vi "UHR-Fleezers Control (host) - 10.3.vi"() -> ()   [LabVIEW 2010] (continued)
          tunnel: w7743 -> [w7751]
          tunnel: w7741 -> [w7750]
          tunnel: w7740 -> [w7749]
          tunnel: [w7748] -> w7739
          tunnel: [w7747] -> w7738
          tunnel: ["Cap 1 Samp Flow ON"] -> w7737
          tunnel: w7739 -> [w7775]
          tunnel: w7738 -> [w7774]
          tunnel: w7737 -> [w7773]
          frame #0 {
            n1615 = local read "Saved Stage Positions"() -> (w7762:dbl[][])
            n1616 = Array Subset(array=w7762, index (row)=0 ("index"), length (row)=1 ("length"), index (col)=1 ("index"), length (col)=3 ("length")) -> (w7759:dbl[][])
            n1617 = Reshape Array(w7759, 3 ("dimension size")) -> (w7757:dbl[])
            n1618 = Array To Cluster(array=w7757) -> (cluster=w7756:cluster{"[0]":dbl, "[1]":dbl, "[2]":dbl})
            n1619 = case shown="True" "Cap 1 Samp Flow ON" {
              tunnel: w7749 -> [w7764 w7770]
              tunnel: w7750 -> [w7765 w7769]
              tunnel: [w7765 w7767] -> w7748
              tunnel: [w7764 w7766] -> w7747
              frame False {
              }
              frame True {
                # "run flow"
                n1620 = Concatenate Strings("run" ("string"), "\r") -> (w7771:string)
                n1621 = VISA Write(VISA resource name=w7769, write buffer=w7771, error in (no error)=w7770) -> (VISA resource name out=w7767:refnum<visa-resource-name>, error out=w7766:errorcluster)  [unwired: 1 out]
              }
            }
            n1622 = call "Set Stage Position.vi"("Position"=w7756, "error in"=w7751, "VISA resource name in"=w7752) -> ("error out"=w7755:errorcluster)  [unwired: 2 out]
            n1623 = local write "Stage Control Serial Error"(w7755) -> ()
            n1624 = local write "Stage Moving"(TRUE ("Stage Moving")) -> ()
          }
          frame #1 {
            n1625 = local write "Stage Moving"(FALSE ("Stage Moving")) -> ()
            n1626 = case shown="True" w7773 {
              tunnel: w7774 -> [w7780 w7786]
              tunnel: w7775 -> [w7781 w7785]
              tunnel: [w7781 w7783] -> _
              tunnel: [w7780 w7782] -> _
              frame False {
              }
              frame True {
                n1627 = Concatenate Strings("stop" ("string"), "\r") -> (w7787:string)
                n1628 = VISA Write(VISA resource name=w7785, write buffer=w7787, error in (no error)=w7786) -> (VISA resource name out=w7783:refnum<visa-resource-name>, error out=w7782:errorcluster)  [unwired: 1 out]
              }
            }
            n1629 = case shown="True" TRUE {
              tunnel: "Cap 1 T ON" -> [w7790 w7791]
              frame False {
                n1630 = property on="Trap 1 (ON/OFF)" class="Bool (strict)"("Val(Sgnl)"=w7790) -> ()  [unwired: 2 in, 2 out]
              }
              frame True {
                n1631 = property on="Trap 2 (ON/OFF)" class="Bool (strict)"("Val(Sgnl)"=w7791) -> ()  [unwired: 2 in, 2 out]
              }
            }
            n1632 = call <vilib>:"Beep.vi"() -> ()  [unwired: 3 in, 9 out]
            n1633 = case shown="True" "Cap 1 Flow ON" {
              frame False {
              }
              frame True {
                n1634 = property on="Inject Pump 1" class="Bool (strict)"("Val(Sgnl)"=TRUE ("Value (Signaling)")) -> ()  [unwired: 2 in, 2 out]
              }
            }
          }
        }
      }
      event "Move Cap. 2 (ADig Left)": Value Change {
        n1635 = event-data() -> ()  [unwired: 1 in, 5 out]
        n1636 = local write "Move Cap. 2 (ADig Left)"(FALSE ("Move Cap. 2 (ADig Left)")) -> ()
        n1637 = flat-sequence {
          tunnel: w7799 -> [w7807]
          tunnel: w7798 -> [w7806]
          tunnel: w7796 -> [w7805]
          tunnel: w7795 -> [w7804]
          tunnel: [w7803] -> w7794
          tunnel: [w7802] -> w7793
          tunnel: ["Cap 2 Samp Flow ON"] -> w7792
          tunnel: w7794 -> [w7830]
          tunnel: w7793 -> [w7829]
          tunnel: w7792 -> [w7828]
          frame #0 {
            n1638 = local read "Saved Stage Positions"() -> (w7817:dbl[][])
            n1639 = case shown="True" "Cap 2 Samp Flow ON" {
              tunnel: w7805 -> [w7819 w7825]
              tunnel: w7804 -> [w7820 w7824]
              tunnel: [w7820 w7822] -> w7803
              tunnel: [w7819 w7821] -> w7802
              frame False {
              }
              frame True {
                # "run flow"
                n1640 = Concatenate Strings("run" ("string"), "\r") -> (w7826:string)
                n1641 = VISA Write(VISA resource name=w7824, write buffer=w7826, error in (no error)=w7825) -> (VISA resource name out=w7822:refnum<visa-resource-name>, error out=w7821:errorcluster)  [unwired: 1 out]
              }
            }
            n1642 = Array Subset(array=w7817, index (row)=1 ("index"), length (row)=1 ("length"), index (col)=1 ("index"), length (col)=3 ("length")) -> (w7814:dbl[][])
            n1643 = Reshape Array(w7814, 3 ("dimension size")) -> (w7812:dbl[])
            n1644 = Array To Cluster(array=w7812) -> (cluster=w7811:cluster{"[0]":dbl, "[1]":dbl, "[2]":dbl})
            n1645 = call "Set Stage Position.vi"("Position"=w7811, "error in"=w7806, "VISA resource name in"=w7807) -> ("error out"=w7810:errorcluster)  [unwired: 2 out]
            n1646 = local write "Stage Moving"(TRUE ("Stage Moving")) -> ()
            n1647 = local write "Stage Control Serial Error"(w7810) -> ()
          }
          frame #1 {
            n1648 = local write "Stage Moving"(FALSE ("Stage Moving")) -> ()
            n1649 = case shown="True" TRUE {
              tunnel: "Cap 2 T ON" -> [w7841 w7842]
              frame False {
                n1650 = property on="Trap 2 (ON/OFF)" class="Bool (strict)"("Val(Sgnl)"=w7841) -> ()  [unwired: 2 in, 2 out]
              }
              frame True {
                n1651 = property on="Trap 1 (ON/OFF)" class="Bool (strict)"("Val(Sgnl)"=w7842) -> ()  [unwired: 2 in, 2 out]
              }
            }
            n1652 = call <vilib>:"Beep.vi"() -> ()  [unwired: 3 in, 9 out]
            n1653 = case shown="True" w7828 {
              tunnel: w7830 -> [_ w7836]
              tunnel: w7829 -> [_ w7835]
              frame False {
              }
              frame True {
                n1654 = Concatenate Strings("stop" ("string"), "\r") -> (w7838:string)
                n1655 = VISA Write(VISA resource name=w7836, write buffer=w7838, error in (no error)=w7835) -> ()  [unwired: 3 out]
              }
            }
            n1656 = case shown="True" "Cap 2 Flow ON" {
              frame False {
              }
              frame True {
                n1657 = property on="Inject Pump 3" class="Bool (strict)"("Val(Sgnl)"=TRUE ("Value (Signaling)")) -> ()  [unwired: 2 in, 2 out]
              }
            }
          }
        }
      }
      event "+z", "-z": Value Change {
        n1658 = event-data() -> ()  [unwired: 1 in, 5 out]
        n1659 = flat-sequence {
          tunnel: w7843 -> [w7865]
          tunnel: w7844 -> [w7845]
          frame #0 {
            n1660 = call "Read Stage Position.vi"("error in"=w7865, "VISA resource name in"=w7845) -> ("Current Position"=w7850:cluster{dbl, dbl, dbl}, "error out"=w7863:errorcluster, "VISA resource name out"=w7864:refnum<visa-resource-name>)  [unwired: 1 out]
            n1661 = local read "Saved Stage Positions"() -> (w7874:dbl[][])
            n1662 = Divide(x="z nudge increment (um)", y=1000.0) -> (x/y=w7862:dbl)
            n1663 = Boolean To (0,1)(Boolean="+z") -> (0, 1=w7854:i16)
            n1664 = Boolean To (0,1)(Boolean="-z") -> (0, 1=w7855:i16)
            n1665 = Array Subset(array=w7874, index (row)=1 ("index"), length (row)=1 ("length"), index (col)=1 ("index"), length (col)=3 ("length")) -> (w7871:dbl[][])
            n1666 = Multiply(x=w7854, y=w7862) -> (x*y=w7858:dbl)
            n1667 = Multiply(x=w7855, y=w7862) -> (x*y=w7856:dbl)
            n1668 = Unbundle(w7850) -> (w7848:dbl, w7847:dbl, w7851:dbl)
            n1669 = Negate(x=w7856) -> (-x=w7857:dbl)
            n1670 = Reshape Array(w7871, 3 ("dimension size")) -> (w7869:dbl[])
            n1671 = Add(x=w7858, y=w7857) -> (x+y=w7859:dbl)
            n1672 = Array To Cluster(array=w7869) -> ()  [unwired: 1 out]
            n1673 = Add(x=w7859, y=w7851) -> (x+y=w7849:dbl)
            n1674 = Bundle(cluster=w7850, w7848, w7847, w7849) -> (w7846:cluster{dbl, dbl, dbl})
            n1675 = call "Set Stage Position.vi"("Position"=w7846, "error in"=w7863, "VISA resource name in"=w7864) -> ("error out"=w7868:errorcluster)  [unwired: 2 out]
            n1676 = local write "Stage Moving"(TRUE ("Stage Moving")) -> ()
            n1677 = local write "Stage Control Serial Error"(w7868) -> ()
          }
          frame #1 {
            n1678 = local write "Stage Moving"(FALSE ("Stage Moving")) -> ()
            n1679 = call <vilib>:"Beep.vi"() -> ()  [unwired: 3 in, 9 out]
          }
        }
      }
      event "Cal/Data Acq. Spot": Value Change {
        # "CALIBRATE DATA ACQUISITION SPOT? LOCATE WHERE TO COLLECT FLUORESCENCE FROM?"
        n1680 = event-data() -> ()  [unwired: 1 in, 5 out]
        n1681 = flat-sequence {
          tunnel: w7880 -> [w7883]
          tunnel: w7879 -> [w7882]
          tunnel: ["Cal @ (MHz)"] -> w7877
          tunnel: w7877 -> [w7903]
          tunnel: w7877 -> [w7924]
          frame #0 {
            n1682 = local read "Saved Stage Positions"() -> (w7886:dbl[][])
            n1683 = Array Subset(array=w7886, index (row)=2 ("index"), length (row)=1 ("length"), index (col)=1 ("index"), length (col)=3 ("length")) -> (w7889:dbl[][])
            n1684 = Reshape Array(w7889, 3 ("dimension size")) -> (w7891:dbl[])
            n1685 = local write "Stage Moving"(TRUE ("Stage Moving")) -> ()
            n1686 = Array To Cluster(array=w7891) -> (cluster=w7892:cluster{"[0]":dbl, "[1]":dbl, "[2]":dbl})
            n1687 = call "Set Stage Position.vi"("Position"=w7892, "error in"=w7882, "VISA resource name in"=w7883) -> ("error out"=w7893:errorcluster)  [unwired: 2 out]
            n1688 = local write "Stage Control Serial Error"(w7893) -> ()
          }
          frame #1 {
            n1689 = property on="Trap Delta (MHz)" class="DigNum (strict)"("Val(Sgnl)"="Cal @ (MHz)") -> ()  [unwired: 2 in, 2 out]
            n1690 = local write "Stage Moving"(FALSE ("Stage Moving")) -> ()
            n1691 = call <vilib>:"Beep.vi"() -> ()  [unwired: 3 in, 9 out]
          }
          frame #2 {
            n1692 = Wait (ms)(milliseconds to wait=u32 100) -> ()  [unwired: 1 out]
          }
          frame #3 {
            n1693 = property on="Save Calibration" class="Bool (strict)"("Val(Sgnl)"=TRUE ("Value (Signaling)")) -> ()  [unwired: 2 in, 2 out]
          }
          frame #4 {
            n1694 = Wait (ms)(milliseconds to wait=u32 4000) -> ()  [unwired: 1 out]
          }
          frame #5 {
            n1695 = while {
              stop <- w7900 stop-if-true
              n1696 = local read "Saving..."() -> (w7901:bool)
              n1697 = Wait (ms)(milliseconds to wait=u32 100) -> ()  [unwired: 1 out]
              n1698 = Not(x=w7901) -> (.not. x?=w7900:bool)
            }
          }
          frame #6 {
            n1699 = case shown="True" "W/ Offset 1" {
              tunnel: w7903 -> [_ w7905]
              frame False {
              }
              frame True {
                n1700 = stacked-sequence {
                  tunnel: w7905 -> [_ _ _ _ _ _ _ w7922]
                  frame #0 {
                    n1701 = property on="Trap Delta (MHz)" class="DigNum (strict)"("Val(Sgnl)"="Offset 1 Start (MHz)") -> ()  [unwired: 2 in, 2 out]
                    n1702 = Replace Array Subset(array=u32[] [0] ("Index Values"), new element="Offset 1 Set", index=0) -> (w7906:u32[])
                    n1703 = property on="Saved AOD Raster Scan Parameter Sets" class="Arr (strict)"("Index Values"=w7906) -> ()  [unwired: 2 in, 2 out]
                  }
                  frame #1 {
                    n1704 = Wait (ms)(milliseconds to wait=u32 200) -> ()  [unwired: 1 out]
                  }
                  frame #2 {
                    n1705 = property on="Load parameters" class="Bool (strict)"("Val(Sgnl)"=TRUE ("Value (Signaling)")) -> ()  [unwired: 2 in, 2 out]
                  }
                  frame #3 {
                    n1706 = Wait (ms)(milliseconds to wait=u32 200) -> ()  [unwired: 1 out]
                  }
                  frame #4 {
                    n1707 = property on="Trap Raster Scan" class="Bool (strict)"("Val(Sgnl)"=TRUE ("Value (Signaling)")) -> ()  [unwired: 2 in, 2 out]
                  }
                  frame #5 {
                    n1708 = Wait (ms)(milliseconds to wait=u32 2000) -> ()  [unwired: 1 out]
                  }
                  frame #6 {
                    n1709 = while {
                      stop <- w7919 stop-if-true
                      n1710 = local read "Raster Scanning..."() -> (w7921:bool)
                      n1711 = local read "Saving..."() -> (w7917:bool)
                      n1712 = Wait (ms)(milliseconds to wait=u32 100) -> ()  [unwired: 1 out]
                      n1713 = Not(x=w7917) -> (.not. x?=w7916:bool)
                      n1714 = Not(x=w7921) -> (.not. x?=w7918:bool)
                      n1715 = And(x=w7918, y=w7916) -> (x .and. y?=w7919:bool)
                    }
                  }
                  frame #7 {
                    n1716 = property on="Trap Delta (MHz)" class="DigNum (strict)"("Val(Sgnl)"=w7922) -> ()  [unwired: 2 in, 2 out]
                  }
                }
              }
            }
          }
          frame #7 {
            n1717 = local read "Save ave N"() -> (w7923:dbl)
            n1718 = case shown="True" "W/ Offset 2" {
              tunnel: w7924 -> [_ w7930]
              tunnel: w7923 -> [_ w7929]
              frame False {
                n1719 = Multiply(x="Cal read wait (s)", y=u32 1000 ("milliseconds to wait")) -> (x*y=w7927:u32)
                n1720 = Wait (ms)(milliseconds to wait=w7927) -> ()  [unwired: 1 out]
              }
              frame True {
                n1721 = stacked-sequence {
                  tunnel: w7930 -> [_ _ _ _ _ _ _ _ _ w7951 _ _]
                  tunnel: w7929 -> [_ _ _ _ _ _ _ _ _ w7949 _ _]
                  frame #0 {
                    n1722 = property on="Save ave N" class="DigNum (strict)"("Val(Sgnl)"=1.0 ("Value (Signaling)")) -> ()  [unwired: 2 in, 2 out]
                  }
                  frame #1 {
                    n1723 = Wait (ms)(milliseconds to wait=u32 500) -> ()  [unwired: 1 out]
                  }
                  frame #2 {
                    n1724 = property on="Trap Delta (MHz)" class="DigNum (strict)"("Val(Sgnl)"="Offset 2 Start (MHz)") -> ()  [unwired: 2 in, 2 out]
                    n1725 = Replace Array Subset(array=u32[] [0] ("Index Values"), new element="Offset 2 Set", index=0) -> (w7935:u32[])
                    n1726 = property on="Saved AOD Raster Scan Parameter Sets" class="Arr (strict)"("Index Values"=w7935) -> ()  [unwired: 2 in, 2 out]
                  }
                  frame #3 {
                    n1727 = Wait (ms)(milliseconds to wait=u32 500) -> ()  [unwired: 1 out]
                  }
                  frame #4 {
                    n1728 = property on="Load parameters" class="Bool (strict)"("Val(Sgnl)"=TRUE ("Value (Signaling)")) -> ()  [unwired: 2 in, 2 out]
                  }
                  frame #5 {
                    n1729 = Wait (ms)(milliseconds to wait=u32 500) -> ()  [unwired: 1 out]
                  }
                  frame #6 {
                    n1730 = property on="Trap Raster Scan" class="Bool (strict)"("Val(Sgnl)"=TRUE ("Value (Signaling)")) -> ()  [unwired: 2 in, 2 out]
                  }
                  frame #7 {
                    n1731 = Wait (ms)(milliseconds to wait=u32 2000) -> ()  [unwired: 1 out]
                  }
                  frame #8 {
                    n1732 = while {
                      stop <- w7944 stop-if-true
                      n1733 = local read "Raster Scanning..."() -> (w7947:bool)
                      n1734 = local read "Saving..."() -> (w7945:bool)
                      n1735 = Wait (ms)(milliseconds to wait=u32 100) -> ()  [unwired: 1 out]
                      n1736 = Not(x=w7945) -> (.not. x?=w7943:bool)
                      n1737 = Not(x=w7947) -> (.not. x?=w7946:bool)
                      n1738 = And(x=w7946, y=w7943) -> (x .and. y?=w7944:bool)
                    }
                  }
                  frame #9 {
                    n1739 = property on="Trap Delta (MHz)" class="DigNum (strict)"("Val(Sgnl)"=w7951) -> ()  [unwired: 2 in, 2 out]
                    n1740 = property on="Saved AOD Raster Scan Parameter Sets" class="Arr (strict)"("Index Values"=u32[] [0]) -> ()  [unwired: 2 in, 2 out]
                    n1741 = property on="Save ave N" class="DigNum (strict)"("Val(Sgnl)"=w7949) -> ()  [unwired: 2 in, 2 out]
                  }
                  frame #10 {
                    n1742 = Wait (ms)(milliseconds to wait=u32 500) -> ()  [unwired: 1 out]
                  }
                  frame #11 {
                    n1743 = property on="Load parameters" class="Bool (strict)"("Val(Sgnl)"=TRUE ("Value (Signaling)")) -> ()  [unwired: 2 in, 2 out]
                  }
                }
              }
            }
          }
          frame #8 {
            n1744 = property on="Read Cal" class="Bool (strict)"("Val(Sgnl)"=TRUE ("Value (Signaling)")) -> ()  [unwired: 2 in, 2 out]
          }
          frame #9 {
            n1745 = Wait (ms)(milliseconds to wait=u32 500) -> ()  [unwired: 1 out]
          }
          frame #10 {
            n1746 = property on="Fish for Tether" class="Bool (strict)"("Val(Sgnl)"=TRUE ("Value (Signaling)")) -> ()  [unwired: 2 in, 2 out]
          }
        }
        n1747 = local write "Cal/Data Acq. Spot"(FALSE ("Cal/Data Acq. Spot")) -> ()
      }
      event "Dump Beads": Value Change {
        # "SCRIPT TO REMOVE BOTH BEADS FROM THE TRAPS. TURNS ON LIGHT WHICH INDICATES THAT STAGE IS MOVING. THEN STOPS SAVING DATA. \nSETS Sample Channel Flow TO TRUE. STOPS INTERLACING GREEN FLUORESCENCE. TURNS OFF Tether INDICATOR BECAUSE WE ARE THROWING IT\nAWAY. SHUTS OFF TRAP POSITION FEEDBACK."
        n1748 = event-data() -> ()  [unwired: 1 in, 5 out]
        n1749 = flat-sequence {
          tunnel: w7958 -> [w7964]
          tunnel: w7957 -> [w7963]
          frame #0 {
            w7960 = FALSE ("Fl. Triggered...")
            w7961 = TRUE ("Stage Moving")
            n1750 = local read "Saving..."() -> (w7962:bool)
            n1751 = local write "Fl. Triggered..."(w7960) -> ()
            n1752 = local write "Stage Moving"(w7961) -> ()
            n1753 = local write "Tether"(w7960) -> ()
            n1754 = property on="Green Laser ON/Interlacing" class="Bool (strict)"("Val(Sgnl)"=w7960) -> ()  [unwired: 2 in, 2 out]
            n1755 = property on="Trap Pos. FB ON" class="Bool (strict)"("Val(Sgnl)"=w7960) -> ()  [unwired: 2 in, 2 out]
            n1756 = property on="Sample Channel Flow" class="Bool (strict)"("Val(Sgnl)"=w7961) -> ()  [unwired: 2 in, 2 out]
            n1757 = local write "Stop Saving"(w7962) -> ()
          }
          frame #1 {
            # "MOVES TO THE DUMP BEADS POSITION"
            n1758 = local read "Saved Stage Positions"() -> (w7965:dbl[][])
            n1759 = Array Subset(array=w7965, index (row)=3 ("index"), length (row)=1 ("length"), index (col)=1 ("index"), length (col)=3 ("length")) -> (w7970:dbl[][])
            n1760 = Reshape Array(w7970, 3 ("dimension size")) -> (w7968:dbl[])
            n1761 = Array To Cluster(array=w7968) -> (cluster=w7967:cluster{"[0]":dbl, "[1]":dbl, "[2]":dbl})
            n1762 = call "Set Stage Position.vi"("Position"=w7967, "error in"=w7963, "VISA resource name in"=w7964) -> ()  [unwired: 3 out]
          }
          frame #2 {
            w7974 = FALSE ("Value (Signaling)")
            # "TURNS TRAPS OFF SO THAT\nBEADS REMAIN AT DUMP \nBEADS POSITION"
            n1763 = property on="Trap 1 (ON/OFF)" class="Bool (strict)"("Val(Sgnl)"=w7974) -> ()  [unwired: 2 in, 2 out]
            n1764 = property on="Trap 2 (ON/OFF)" class="Bool (strict)"("Val(Sgnl)"=w7974) -> ()  [unwired: 2 in, 2 out]
            n1765 = call <vilib>:"Beep.vi"() -> ()  [unwired: 3 in, 9 out]
          }
          frame #3 {
            # "MOVES STAGE BACK TO THE\nANTIDIG CAPILARY BY CALLING\nTHE Move Cap. 2 SCRIPT"
            n1766 = property on="Move Cap. 2 (ADig Left)" class="Bool (strict)"("Val(Sgnl)"=TRUE ("Value (Signaling)")) -> ()  [unwired: 2 in, 2 out]
          }
        }
      }
      event "Dip for Protein": Value Change {
        n1767 = event-data() -> ()  [unwired: 1 in, 5 out]
        n1768 = flat-sequence {
          tunnel: w7982 -> [w7986]
          tunnel: w7983 -> [w7987]
          tunnel: [w7987] -> w7977
          tunnel: [w7986] -> w7976
          tunnel: [w7990] -> w7980
          tunnel: [w7989] -> w7978
          tunnel: w7977 -> [w7993]
          tunnel: w7976 -> [w7992]
          tunnel: [w8003] -> w7981
          tunnel: w7980 -> [w8003]
          tunnel: [w8002] -> w7979
          tunnel: w7978 -> [w8002]
          tunnel: w7981 -> [w8008]
          tunnel: w7979 -> [w8007]
          frame #0 {
            n1769 = case shown="True" "Move Trap Before?" {
              frame False {
              }
              frame True {
                n1770 = property on="Trap Delta (MHz)" class="DigNum (strict)"("Val(Sgnl)"="Dip Trap Delta 1 (MHz)") -> ()  [unwired: 2 in, 2 out]
              }
            }
          }
          frame #1 {
            n1771 = local read "Saved Stage Positions"() -> (w7991:dbl[][])
            n1772 = Array Subset(array=w7991, index (row)=4 ("index"), length (row)=1 ("length"), index (col)=1 ("index"), length (col)=3 ("length")) -> (w7998:dbl[][])
            n1773 = Reshape Array(w7998, 3 ("dimension size")) -> (w7996:dbl[])
            n1774 = Array To Cluster(array=w7996) -> (cluster=w7995:cluster{"[0]":dbl, "[1]":dbl, "[2]":dbl})
            n1775 = call "Set Stage Position.vi"("Position"=w7995, "error in"=w7992, "VISA resource name in"=w7993) -> ("error out"=w7989:errorcluster, "VISA resource name out"=w7990:refnum<visa-resource-name>)  [unwired: 1 out]
          }
          frame #2 {
            n1776 = Multiply(x="Duration (s)", y=1000.0) -> (x*y=w8004:dbl)
            n1777 = Wait (ms)(milliseconds to wait=w8004) -> ()  [unwired: 1 out]
          }
          frame #3 {
            n1778 = local read "Saved Stage Positions"() -> (w8009:dbl[][])
            n1779 = Array Subset(array=w8009, index (row)=2 ("index"), length (row)=1 ("length"), index (col)=1 ("index"), length (col)=3 ("length")) -> (w8014:dbl[][])
            n1780 = Reshape Array(w8014, 3 ("dimension size")) -> (w8012:dbl[])
            n1781 = Array To Cluster(array=w8012) -> (cluster=w8011:cluster{"[0]":dbl, "[1]":dbl, "[2]":dbl})
            n1782 = call "Set Stage Position.vi"("Position"=w8011, "error in"=w8007, "VISA resource name in"=w8008) -> ()  [unwired: 3 out]
          }
          frame #4 {
            n1783 = case shown="True" "Move Trap After?" {
              frame False {
              }
              frame True {
                n1784 = property on="Trap Delta (MHz)" class="DigNum (strict)"("Val(Sgnl)"="Dip Trap Delta 2 (MHz)") -> ()  [unwired: 2 in, 2 out]
              }
            }
          }
          frame #5 {
            n1785 = case shown="True" "Green ON After?" {
              frame False {
              }
              frame True {
                n1786 = property on="Green Laser ON/Interlacing" class="Bool (strict)"("Val(Sgnl)"=TRUE ("Value (Signaling)")) -> ()  [unwired: 2 in, 2 out]
              }
            }
          }
          frame #6 {
            n1787 = Wait (ms)(milliseconds to wait=u32 500) -> ()  [unwired: 1 out]
          }
          frame #7 {
            n1788 = case shown="True" "Save Data After?" {
              frame False {
              }
              frame True {
                n1789 = property on="Start Saving" class="Bool (strict)"("Val(Sgnl)"=TRUE ("Value (Signaling)")) -> ()  [unwired: 2 in, 2 out]
              }
            }
          }
        }
      }
      event "Profile": Value Change {
        n1790 = event-data() -> ()  [unwired: 1 in, 5 out]
        n1791 = flat-sequence {
          tunnel: w8033 -> [w8036]
          tunnel: w8032 -> [w8044]
          tunnel: [w8038] -> w8031
          tunnel: [w8037] -> w8030
          tunnel: [w8035] -> w8028
          tunnel: [w8034] -> w8025
          tunnel: w8031 -> [w8051]
          tunnel: w8030 -> [w8050]
          tunnel: [w8048] -> w8029
          tunnel: w8028 -> [w8049]
          tunnel: [w8047] -> w8027
          tunnel: [w8046] -> w8026
          tunnel: w8025 -> [w8046]
          tunnel: w8029 -> [w8055]
          tunnel: w8027 -> [w8054]
          tunnel: w8026 -> [w8053]
          frame #0 {
            n1792 = call "Read Stage Position.vi"("error in"=w8044, "VISA resource name in"=w8036) -> ("Current Position"=w8034:cluster{dbl, dbl, dbl}, "error out"=w8037:errorcluster, "VISA resource name out"=w8035:refnum<visa-resource-name>)  [unwired: 1 out]
            "Current Position" <- w8034
            n1793 = local write "Stage Control Serial Error"(w8037) -> ()
            n1794 = Unbundle(w8034) -> (w8041:dbl, w8043:dbl, w8039:dbl)
            n1795 = Add(x=w8043, y="Y change (mm)") -> (x+y=w8040:dbl)
            n1796 = Bundle(w8041, w8040, w8039) -> (w8038:cluster{dbl, dbl, dbl})  [unwired: 1 in]
          }
          frame #1 {
            # "move to new position and start saving"
            n1797 = local write "Stage Moving"(TRUE ("Stage Moving")) -> ()
            n1798 = local write "Start Saving"(TRUE ("Start Saving")) -> ()
            n1799 = call "Set Stage Position.vi"("Position"=w8051, "error in"=w8050, "VISA resource name in"=w8049) -> ("error out"=w8047:errorcluster, "VISA resource name out"=w8048:refnum<visa-resource-name>)  [unwired: 1 out]
          }
          frame #2 {
            # "go back to start"
            n1800 = call "Set Stage Position.vi"("Position"=w8053, "error in"=w8054, "VISA resource name in"=w8055) -> ()  [unwired: 3 out]
          }
          frame #3 {
            # "stop saving"
            n1801 = local write "Stop Saving"(TRUE ("Stop Saving")) -> ()
            n1802 = local write "Stage Moving"(FALSE ("Stage Moving")) -> ()
          }
        }
      }
      event "Move to Position 1", "Move to Position 2", "Move to Position 3", "Move to Position 4", "Move to Position 5", "Lower Ch. Cap.": Value Change {
        n1803 = event-data() -> ()  [unwired: 1 in, 5 out]
        n1804 = Or(x="Move to Position 5", y="Lower Ch. Cap.") -> (x .or. y?=w8061:bool)
        n1805 = Build Array("Move to Position 1", "Move to Position 2", "Move to Position 3", "Move to Position 4", w8061) -> (w8064:bool[])
        n1806 = Boolean Array To Number(Boolean array=w8064) -> (number=w8063:u32)
        n1807 = Logarithm Base 2(1:w8063) -> (0:w8062:dbl)
        n1808 = flat-sequence {
          tunnel: w8062 -> [w8073]
          tunnel: w8059 -> [w8071]
          tunnel: w8058 -> [w8070]
          frame #0 {
            n1809 = local read "Saved Stage Positions"() -> (w8081:dbl[][])
            n1810 = Array Subset(array=w8081, index (row)=w8073, length (row)=1 ("length"), index (col)=1 ("index"), length (col)=3 ("length")) -> (w8078:dbl[][])
            n1811 = Reshape Array(w8078, 3 ("dimension size")) -> (w8076:dbl[])
            n1812 = Array To Cluster(array=w8076) -> (cluster=w8075:cluster{"[0]":dbl, "[1]":dbl, "[2]":dbl})
            n1813 = call "Set Stage Position.vi"("Position"=w8075, "error in"=w8070, "VISA resource name in"=w8071) -> ("error out"=w8074:errorcluster)  [unwired: 2 out]
            n1814 = local write "Stage Moving"(TRUE ("Stage Moving")) -> ()
            n1815 = local write "Stage Control Serial Error"(w8074) -> ()
          }
          frame #1 {
            n1816 = local write "Stage Moving"(FALSE ("Stage Moving")) -> ()
            n1817 = call <vilib>:"Beep.vi"() -> ()  [unwired: 3 in, 9 out]
          }
        }
      }
      event "Got ADig bead": Value Change {
        n1818 = event-data() -> ()  [unwired: 1 in, 5 out]
        n1819 = property on="Move Cap. 1 (DNA Right)" class="Bool (strict)"("Val(Sgnl)"=TRUE ("Value (Signaling)")) -> ()  [unwired: 2 in, 2 out]
        n1820 = property on="Inject Pump 3" class="Bool (strict)"("Val(Sgnl)"=FALSE ("Value (Signaling)")) -> ()  [unwired: 2 in, 2 out]
      }
      event "Got DNA bead": Value Change {
        n1821 = event-data() -> ()  [unwired: 1 in, 5 out]
        n1822 = property on="Cal/Data Acq. Spot" class="Bool (strict)"("Val(Sgnl)"=TRUE ("Value (Signaling)")) -> ()  [unwired: 2 in, 2 out]
        n1823 = property on="Inject Pump 1" class="Bool (strict)"("Val(Sgnl)"=FALSE ("Value (Signaling)")) -> ()  [unwired: 2 in, 2 out]
      }
      event "Take Stepping Data": Value Change {
        n1824 = event-data() -> ()  [unwired: 1 in, 5 out]
        n1825 = local read "Save ave N"() -> (w8098:dbl)
        n1826 = flat-sequence {
          tunnel: w8098 -> [w8100]
          tunnel: [w8100] -> w8093
          tunnel: [w8102] -> w8094
          tunnel: w8093 -> [w8102]
          tunnel: [w8104] -> w8095
          tunnel: w8094 -> [w8104]
          tunnel: [w8107] -> w8096
          tunnel: w8095 -> [w8107]
          tunnel: [w8109] -> w8097
          tunnel: w8096 -> [w8109]
          tunnel: [w8111] -> w8091
          tunnel: w8097 -> [w8111]
          tunnel: w8091 -> [w8114]
          tunnel: [w8114] -> w8090
          tunnel: w8090 -> [w8115]
          tunnel: [w8115] -> w8092
          tunnel: w8092 -> [w8121]
          frame #0 {
            n1827 = property on="Save ave N" class="DigNum (strict)"("Val(Sgnl)"="Save ave factor") -> ()  [unwired: 2 in, 2 out]
          }
          frame #1 {
            n1828 = Wait (ms)(milliseconds to wait=u32 100) -> ()  [unwired: 1 out]
          }
          frame #2 {
            n1829 = local read "Offset 2 Start (MHz)"() -> (w8106:dbl)
            n1830 = property on="Saved AOD Raster Scan Parameter Sets" class="Arr (strict)"("Index Values"=u32[] [2]) -> ()  [unwired: 2 in, 2 out]
            n1831 = property on="Trap Delta (MHz)" class="DigNum (strict)"("Val(Sgnl)"=w8106) -> ()  [unwired: 2 in, 2 out]
          }
          frame #3 {
            n1832 = property on="Load parameters" class="Bool (strict)"("Val(Sgnl)"=TRUE ("Value (Signaling)")) -> ()  [unwired: 2 in, 2 out]
          }
          frame #4 {
            n1833 = Wait (ms)(milliseconds to wait=u32 100) -> ()  [unwired: 1 out]
          }
          frame #5 {
            n1834 = property on="Trap Raster Scan" class="Bool (strict)"("Val(Sgnl)"=TRUE ("Value (Signaling)")) -> ()  [unwired: 2 in, 2 out]
          }
          frame #6 {
            n1835 = Wait (ms)(milliseconds to wait=u32 1000) -> ()  [unwired: 1 out]
          }
          frame #7 {
            n1836 = while {
              stop <- w8118 stop-if-true
              n1837 = local read "Raster Scanning..."() -> (w8120:bool)
              n1838 = local read "Saving..."() -> (w8119:bool)
              n1839 = Not(x=w8119) -> (.not. x?=w8116:bool)
              n1840 = Not(x=w8120) -> (.not. x?=w8117:bool)
              n1841 = And(x=w8117, y=w8116) -> (x .and. y?=w8118:bool)
            }
          }
          frame #8 {
            n1842 = property on="Save ave N" class="DigNum (strict)"("Val(Sgnl)"=w8121) -> ()  [unwired: 2 in, 2 out]
          }
        }
      }
      event "Step Size (nm)": Value Change {
        n1843 = event-data() -> ()  [unwired: 1 in, 5 out]
        n1844 = flat-sequence {
          frame #0 {
            n1845 = property on="Saved AOD Raster Scan Parameter Sets" class="Arr (strict)"("Index Values"=u32[] [1]) -> ()  [unwired: 2 in, 2 out]
          }
          frame #1 {
            n1846 = Multiply(x="N Steps", y="Step Size (nm)") -> (x*y=w8123:dbl)
            n1847 = property on="Scan Speed AOD (nm/s) 2" class="DigNum (strict)"("Value"="Step Size (nm)") -> ()  [unwired: 2 in, 2 out]
            n1848 = property on="Step Size AOD (nm) 2" class="DigNum (strict)"("Value"="Step Size (nm)") -> ()  [unwired: 2 in, 2 out]
            n1849 = property on="Scan Range AOD (nm) 2" class="DigNum (strict)"("Value"=w8123) -> ()  [unwired: 2 in, 2 out]
          }
        }
      }
      event "Take Detection Laser\nImage": Value Change {
        n1850 = event-data() -> ()  [unwired: 1 in, 5 out]
        n1851 = flat-sequence {
          tunnel: [w8151] -> w8141
          tunnel: [w8150] -> w8134
          tunnel: [w8149] -> w8126
          tunnel: [w8154] -> w8142
          tunnel: w8141 -> [w8154]
          tunnel: [w8153] -> w8135
          tunnel: w8134 -> [w8153]
          tunnel: [w8152] -> w8127
          tunnel: w8126 -> [w8152]
          tunnel: [w8158] -> w8143
          tunnel: w8142 -> [w8158]
          tunnel: [w8157] -> w8136
          tunnel: w8135 -> [w8157]
          tunnel: [w8156] -> w8128
          tunnel: w8127 -> [w8156]
          tunnel: [w8164] -> w8144
          tunnel: w8143 -> [w8164]
          tunnel: [w8163] -> w8137
          tunnel: w8136 -> [w8163]
          tunnel: [w8162] -> w8129
          tunnel: w8128 -> [w8162]
          tunnel: [w8168] -> w8145
          tunnel: w8144 -> [w8168]
          tunnel: [w8167] -> w8138
          tunnel: w8137 -> [w8167]
          tunnel: [w8166] -> w8130
          tunnel: w8129 -> [w8166]
          tunnel: [w8172] -> w8146
          tunnel: w8145 -> [w8172]
          tunnel: [w8171] -> w8139
          tunnel: w8138 -> [w8171]
          tunnel: [w8170] -> w8131
          tunnel: w8130 -> [w8170]
          tunnel: [w8176] -> w8147
          tunnel: w8146 -> [w8176]
          tunnel: [w8175] -> w8140
          tunnel: w8139 -> [w8175]
          tunnel: [w8174] -> w8132
          tunnel: w8131 -> [w8174]
          tunnel: w8147 -> [w8182]
          tunnel: w8140 -> [w8181]
          tunnel: [w8179] -> w8133
          tunnel: w8132 -> [w8179]
          tunnel: w8133 -> [w8183]
          frame #0 {
            n1852 = local read "Green Laser ON/Interlacing"() -> (w8151:bool)
            n1853 = local read "Green laser mode"() -> (w8150:enum32{"Laser ON", "Laser OFF", "Interlace"})
            n1854 = local read "Green FB On/Off"() -> (w8149:bool)
          }
          frame #1 {
            n1855 = property on="Green FB On/Off" class="Bool (strict)"("Val(Sgnl)"=FALSE ("Value (Signaling)")) -> ()  [unwired: 2 in, 2 out]
          }
          frame #2 {
            n1856 = property on="Green Laser ON/Interlacing" class="Bool (strict)"("Val(Sgnl)"=TRUE ("Value (Signaling)")) -> ()  [unwired: 2 in, 2 out]
            n1857 = property on="Flip Green Filter" class="Bool (strict)"("Val(Sgnl)"=TRUE ("Value (Signaling)")) -> ()  [unwired: 2 in, 2 out]
            n1858 = property on="Green laser mode" class="RadioBtnsControl (strict)"("Val(Sgnl)"=enum32{"Laser ON", "Laser OFF", "Interlace"}."Laser ON" ("Value (Signaling)")) -> ()  [unwired: 2 in, 2 out]
          }
          frame #3 {
            n1859 = Wait (ms)(milliseconds to wait=u32 500) -> ()  [unwired: 1 out]
          }
          frame #4 {
            n1860 = property on="Confocal Image" class="Bool (strict)"("Val(Sgnl)"=TRUE ("Value (Signaling)")) -> ()  [unwired: 2 in, 2 out]
          }
          frame #5 {
            n1861 = Wait (ms)(milliseconds to wait=u32 2000) -> ()  [unwired: 1 out]
          }
          frame #6 {
            n1862 = while {
              stop <- w8177 stop-if-true
              n1863 = local read "Saving..."() -> (w8178:bool)
              n1864 = Not(x=w8178) -> (.not. x?=w8177:bool)
            }
          }
          frame #7 {
            n1865 = property on="Flip Green Filter" class="Bool (strict)"("Val(Sgnl)"=TRUE ("Value (Signaling)")) -> ()  [unwired: 2 in, 2 out]
            n1866 = property on="Green Laser ON/Interlacing" class="Bool (strict)"("Val(Sgnl)"=w8182) -> ()  [unwired: 2 in, 2 out]
            n1867 = property on="Green laser mode" class="RadioBtnsControl (strict)"("Val(Sgnl)"=w8181) -> ()  [unwired: 2 in, 2 out]
          }
          frame #8 {
            n1868 = property on="Green FB On/Off" class="Bool (strict)"("Val(Sgnl)"=w8183) -> ()  [unwired: 2 in, 2 out]
          }
        }
      }
      event "Stop All": Value Change {
        n1869 = event-data() -> ()  [unwired: 1 in, 5 out]
        n1870 = local read "Stop All"() -> (w8184:bool)
      }
    }
    n1871 = node-c288() -> ()  [unwired: 1 in, 1 out]
  }
  n1872 = timed-loop "Mouse control: trap position (AOM deflection), set confocal spot from image" {
    tunnel: [w8186] -> w155
    tunnel: w8 -> [w8185]
    timing: w51 -> [_]
    timing-out: [_] -> w50
    stop <- w8186 stop-if-true
    n1873 = node-c288() -> ()  [unwired: 2 out]
    n1874 = event shown="[0] \"Pane\": Mouse Down" {
      selector: _ -> [_ _]
      dyn-events: _ -> [_ _]
      timeout: _ -> [_ _]
      tunnel: w8185 -> [w8189 _]
      event Mouse Down {
        n1875 = event-data() -> ("Time"=w8191:u32, "Coords"=w8190:T7, "Button"=w8192:u16)  [unwired: 6 out]
        n1876 = case shown="3" w8192 {
          tunnel: w8191 -> [_ _ w8295]
          tunnel: w8190 -> [_ w8229 w8293]
          tunnel: w8189 -> [_ _ w8291]
          frame 0, Default {
          }
          frame 1 {
            n1877 = property on="APD 2" class="ImageControl"() -> ("Displayed Image Position"=w8199:cluster{"Left":i32, "Top":i32})  [unwired: 2 in, 2 out]
            n1878 = property on="APD 1" class="ImageControl"() -> ("Displayed Image Position"=w8228:cluster{"Left":i32, "Top":i32})  [unwired: 2 in, 2 out]
            n1879 = property on="Detection Laser X" class="ImageControl"() -> ("Displayed Image Position"=w8225:cluster{"Left":i32, "Top":i32})  [unwired: 2 in, 2 out]
            n1880 = property on="Detection Laser Y" class="ImageControl"() -> ("Displayed Image Position"=w8224:cluster{"Left":i32, "Top":i32})  [unwired: 2 in, 2 out]
            n1881 = property on="APD 2" class="ImageControl"() -> ("Displayed Image Size"=w8198:cluster{"Width":u32, "Height":u32})  [unwired: 2 in, 2 out]
            n1882 = property on="APD 1" class="ImageControl"() -> ("Displayed Image Size"=w8226:cluster{"Width":u32, "Height":u32})  [unwired: 2 in, 2 out]
            n1883 = property on="Detection Laser X" class="ImageControl"() -> ("Displayed Image Size"=w8227:cluster{"Width":u32, "Height":u32})  [unwired: 2 in, 2 out]
            n1884 = property on="Detection Laser Y" class="ImageControl"() -> ("Displayed Image Size"=w8223:cluster{"Width":u32, "Height":u32})  [unwired: 2 in, 2 out]
            n1885 = Unbundle By Name(w8198) -> ("Width"=w8195:u32, "Height"=w8194:u32)
            n1886 = Unbundle By Name(w8199) -> ("Left"=w8197:i32, "Top"=w8196:i32)
            n1887 = Unbundle By Name(w8226) -> ("Width"=w8220:u32, "Height"=w8219:u32)
            n1888 = Unbundle By Name(w8227) -> ("Width"=w8216:u32, "Height"=w8215:u32)
            n1889 = Unbundle By Name(w8223) -> ("Width"=w8212:u32, "Height"=w8211:u32)
            n1890 = Unbundle By Name(w8228) -> ("Left"=w8222:i32, "Top"=w8221:i32)
            n1891 = Unbundle By Name(w8225) -> ("Left"=w8218:i32, "Top"=w8217:i32)
            n1892 = Unbundle By Name(w8224) -> ("Left"=w8214:i32, "Top"=w8213:i32)
            n1893 = Bundle("Left"=w8197, "Top"=w8196, "Width"=w8195, "Height"=w8194) -> (w8193:T45)  [unwired: 1 in]
            n1894 = Bundle("Left"=w8222, "Top"=w8221, "Width"=w8220, "Height"=w8219) -> (w8210:T45)  [unwired: 1 in]
            n1895 = Bundle("Left"=w8218, "Top"=w8217, "Width"=w8216, "Height"=w8215) -> (w8209:T45)  [unwired: 1 in]
            n1896 = Bundle("Left"=w8214, "Top"=w8213, "Width"=w8212, "Height"=w8211) -> (w8208:T45)  [unwired: 1 in]
            n1897 = Build Cluster Array(w8193, w8210, w8209, w8208) -> (w8207:T46)
            n1898 = for {
              tunnel: w8229 -> [w8240]
              tunnel: w8207 -> [w8241] mode=indexing
              shift-right: [w8238] -> w8205
              shift-left: TRUE -> [w8239]
              shift-right: [w8237] -> w8203
              shift-left: _ -> [w8233]
              shift-right: [w8236] -> w8202
              shift-left: _ -> [w8232]
              shift-right: [w8235] -> w8201
              shift-left: _ -> [w8231]
              shift-right: [w8234] -> w8200
              shift-left: _ -> [w8230]
              n1899 = case shown="True" w8239 {
                selector: w8239 -> [w8246 _]
                tunnel: w8241 -> [_ w8255]
                tunnel: w8240 -> [_ w8253]
                tunnel: [w8246 w8251] -> w8238
                tunnel: [w8245 w8250] -> w8237
                tunnel: [w8244 w8249] -> w8236
                tunnel: [w8243 w8248] -> w8235
                tunnel: [w8242 w8247] -> w8234
                tunnel: w8233 -> [w8245 _]
                tunnel: w8232 -> [w8244 _]
                tunnel: w8231 -> [w8243 _]
                tunnel: w8230 -> [w8242 _]
                frame False {
                }
                frame True {
                  n1900 = Unbundle(w8255) -> (w8254:T45)
                  n1901 = call "isclickinwindow.vi"("Image Param"=w8254, "Point32"=w8253) -> ("4 Y"=w8247:i32, "3 Height"=w8248:i32, "2 X"=w8249:i32, "1 Width"=w8250:i32, "In image?"=w8252:bool)  [unwired: 1 in]
                  n1902 = Not(x=w8252) -> (.not. x?=w8251:bool)
                }
              }
            }
            n1903 = Not(x=w8205) -> (.not. x?=w8204:bool)
            n1904 = case shown="True" w8204 {
              tunnel: w8202 -> [_ w8268]
              tunnel: w8200 -> [_ w8267]
              tunnel: w8203 -> [_ w8266]
              tunnel: w8201 -> [_ w8265]
              frame False {
              }
              frame True {
                w8261 = FALSE ("Get Point")
                n1905 = local read "Scan lines (y)"() -> (w8270:u64)
                n1906 = local read "Actual MCL Inc (V)"() -> (w8262:dbl)
                n1907 = local read "Scan steps (MCL)"() -> (w8269:u64)
                n1908 = Divide "Y Pix/step"(x=w8265, y=w8270) -> (x/y=w8277:dbl)
                n1909 = Divide "Y V/pix"(x=w8262, y=w8277) -> (x/y=w8276:dbl)
                n1910 = Divide "Y half step offset"(x=w8262, y=2.0) -> (x/y=w8278:dbl)
                n1911 = Divide "X pix/step"(x=w8266, y=w8269) -> (x/y=w8275:dbl)
                n1912 = Negate(x=w8278) -> (-x=w8279:dbl)
                n1913 = local read "Initial Y"() -> (w8285:dbl)
                n1914 = Multiply(x=w8267, y=w8276) -> (x*y=w8286:dbl)
                n1915 = Divide "X half step offset"(x=w8262, y=2.0) -> (x/y=w8272:dbl)
                n1916 = Divide "X V/pix"(x=w8262, y=w8275) -> (x/y=w8274:dbl)
                n1917 = Multiply(x=w8262, y=w8269) -> (x*y=w8281:dbl)
                n1918 = Compound Arithmetic op=ADD(w8279, w8286, w8285) -> (w8263:dbl)
                "Pointer Y (V)" <- w8263
                n1919 = Multiply(x=w8274, y=w8268) -> (x*y=w8283:dbl)
                n1920 = Negate(x=w8272) -> (-x=w8271:dbl)
                n1921 = local read "Initial X"() -> (w8284:dbl)
                n1922 = Negate(x=w8283) -> (-x=w8282:dbl)
                n1923 = Compound Arithmetic op=ADD(w8271, w8281, w8284, w8282) -> (w8264:dbl)
                "Pointer X (V)" <- w8264
                n1924 = Or(x="Set X Only", y="Set Confocal Spot (X-Y)") -> (x .or. y?=w8257:bool)
                n1925 = Or(x="Set Confocal Spot (X-Y)", y="Set Y Only") -> (x .or. y?=w8256:bool)
                n1926 = case shown="True" w8257 {
                  tunnel: w8264 -> [_ w8287]
                  frame False {
                  }
                  frame True {
                    n1927 = property on="AO2" class="Slide (strict)"("Val(Sgnl)"=w8287) -> ()  [unwired: 2 in, 2 out]
                  }
                }
                n1928 = case shown="True" w8256 {
                  tunnel: w8263 -> [_ w8288]
                  frame False {
                  }
                  frame True {
                    n1929 = property on="AO1" class="Slide (strict)"("Val(Sgnl)"=w8288) -> ()  [unwired: 2 in, 2 out]
                  }
                }
                n1930 = local write "Set Confocal Spot (X-Y)"(w8261) -> ()
                n1931 = local write "Set X Only"(w8261) -> ()
                n1932 = local write "Set Y Only"(w8261) -> ()
              }
            }
          }
          frame 3 {
            n1933 = local read "BD 2 Frequency 1 (MHz)"() -> (w8289:dbl)
            n1934 = local read "BD 1 Frequency 1 (MHz)"() -> (w8290:dbl)
            n1935 = local write "Manipulating Trap"(TRUE ("Manipulating Trap")) -> ()
            n1936 = local write "Coords"(T7 {"Horizontal"=0, "Vertical"=0} ("Coords")) -> ()
            n1937 = while {
              tunnel: w8295 -> [w8300]
              tunnel: w8293 -> [w8299]
              tunnel: w8291 -> [w8298]
              tunnel: w8290 -> [w8297]
              tunnel: w8289 -> [w8296]
              stop <- w8301 stop-if-true
              n1938 = event shown="[0] \"Pane\": Mouse Move" {
                selector: _ -> [_ _]
                dyn-events: _ -> [_ _]
                timeout: _ -> [_ _]
                tunnel: ["Force Manip Abort" w8365] -> w8301
                tunnel: w8300 -> [w8308 _]
                tunnel: w8299 -> [w8306 _]
                tunnel: w8298 -> [w8305 _]
                tunnel: w8297 -> [w8304 _]
                tunnel: w8296 -> [w8303 _]
                event Mouse Move {
                  n1939 = event-data() -> ("Time"=w8309:u32, "Coords"=w8310:T7)  [unwired: 3 out]
                  n1940 = Less?(x=w8309, y=w8308) -> (x < y?=w8307:bool)
                  n1941 = case "Makes sure old motion events prior to mouse click aren't used" shown="False" w8307 {
                    tunnel: w8310 -> [w8352 _]
                    tunnel: w8306 -> [w8353 _]
                    tunnel: w8305 -> [w8330 _]
                    tunnel: w8304 -> [w8326 _]
                    tunnel: w8303 -> [w8325 _]
                    frame False {
                      n1942 = Subtract(x=w8352, y=w8353) -> (x-y=w8351:T7)
                      "Coords" <- w8351
                      n1943 = local read "Y RF Frequency Limits (MHz)"() -> (w8311:T16)
                      n1944 = To Double Precision Float(number=w8351) -> (double precision float=w8350:cluster{"Horizontal":dbl, "Vertical":dbl})
                      n1945 = Multiply(x=cluster{"Horizontal":dbl, "Vertical":dbl} {"Horizontal"=-1.0, "Vertical"=1.0}, y="Manipulation Scaling") -> (x*y=w8346:cluster{"Horizontal":dbl, "Vertical":dbl})
                      n1946 = local read "X RF Frequency Limits (MHz)"() -> (w8312:T16)
                      n1947 = Multiply(x=w8350, y=w8346) -> (x*y=w8348:cluster{"Horizontal":dbl, "Vertical":dbl})
                      n1948 = Unbundle By Name(w8348) -> ("Horizontal"=w8343:dbl, "Vertical"=w8347:dbl)
                      n1949 = Unbundle By Name(w8311) -> ("Maximum"=w8314:dbl, "Minimum"=w8313:dbl)
                      n1950 = Boolean To (0,1)(Boolean="Manip. X?") -> (0, 1=w8341:i16)
                      n1951 = Boolean To (0,1)(Boolean="Manip. Y?") -> (0, 1=w8338:i16)
                      n1952 = local read "BD 1 Frequency 2 (MHz)"() -> (w8328:dbl)
                      n1953 = Multiply(x=w8347, y=w8338) -> (x*y=w8340:dbl)
                      n1954 = Multiply(x=w8341, y=w8343) -> (x*y=w8344:dbl)
                      n1955 = local read "BD 2 Frequency 2 (MHz)"() -> (w8327:dbl)
                      n1956 = Unbundle By Name(w8312) -> ("Maximum"=w8316:dbl, "Minimum"=w8315:dbl)
                      n1957 = Add(x=w8325, y=w8340) -> (x+y=w8318:dbl)
                      n1958 = Add(x=w8326, y=w8344) -> (x+y=w8320:dbl)
                      n1959 = In Range and Coerce(upper limit=w8316, x=w8320, lower limit=w8315) -> (coerced(x)=w8319:dbl)  [unwired: 1 out]
                      n1960 = In Range and Coerce(upper limit=w8314, x=w8318, lower limit=w8313) -> (coerced(x)=w8317:dbl)  [unwired: 1 out]
                      n1961 = Subtract(x=w8319, y=w8328) -> (x-y=w8337:dbl)
                      n1962 = Subtract(x=w8317, y=w8327) -> (x-y=w8336:dbl)
                      n1963 = Square(x=w8337) -> (x^2=w8335:dbl)
                      n1964 = Square(x=w8336) -> (x^2=w8334:dbl)
                      n1965 = Add(x=w8335, y=w8334) -> (x+y=w8333:dbl)
                      n1966 = Square Root(x=w8333) -> (sqrt(x)=w8329:dbl)
                      n1967 = In Range and Coerce(upper limit="Limit Max (MHz)", x=w8329, lower limit="Limit Min (MHz)") -> (In Range?=w8322:bool)  [unwired: 1 out]
                      n1968 = Not(x="Limits Enable") -> (.not. x?=w8321:bool)
                      n1969 = Or(x=w8322, y=w8321) -> (x .or. y?=w8323:bool)
                      n1970 = case shown="True" w8323 {
                        tunnel: w8330 -> [_ w8363]
                        tunnel: w8329 -> [_ w8354]
                        tunnel: w8319 -> [_ w8361]
                        tunnel: w8328 -> [_ w8360]
                        tunnel: w8317 -> [_ w8359]
                        tunnel: w8327 -> [_ w8358]
                        tunnel: w8312 -> [_ w8356]
                        tunnel: w8311 -> [_ w8355]
                        frame False {
                        }
                        frame True {
                          n1971 = local read "BD 1 Frequency 3 (MHz)"() -> (w8362:dbl)
                          n1972 = local read "BD 2 Frequency 3 (MHz)"() -> (w8357:dbl)
                          n1973 = local write "Trap Delta (MHz)"(w8354) -> ()
                          n1974 = property on="Initial delta (MHz)" class="DigNum (strict)"("Val(Sgnl)"=w8354) -> ()  [unwired: 2 in, 2 out]
                          n1975 = call "set RF board frequency - interlace.vi"("Board 2 Frequency Limits"=w8355, "Board 1 Frequency Limits"=w8356, "FPGA VI Reference In"=w8363, "Board 2 Frequency 3 (MHz)"=w8357, "Board 1 Frequency 3 (MHz)"=w8362, "Board 2 Frequency 2 (MHz)"=w8358, "Board 2 Frequency 1 (MHz)"=w8359, "Board 1 Frequency 2 (MHz)"=w8360, "Board 1 Frequency 1  (MHz)"=w8361) -> ()  [unwired: 1 in, 2 out]